vi "Dresden R2R Sputter 03.02.2018 IY24.vi"() -> ()   [LabVIEW 2009] (continued)
        n1597 = In Range and Coerce(upper limit=1002, x=w2926, lower limit=965) -> (In Range?=w3115:bool)  [unwired: 1 out]
        n1598 = In Range and Coerce(upper limit=679, x=w2926, lower limit=640) -> (In Range?=w3110:bool)  [unwired: 1 out]
        n1599 = In Range and Coerce(upper limit=475, x=w2926, lower limit=441) -> (In Range?=w3081:bool)  [unwired: 1 out]
        n1600 = In Range and Coerce(upper limit=115, x=w2925, lower limit=31) -> (In Range?=w3449:bool)  [unwired: 1 out]
        n1601 = In Range and Coerce(upper limit=537, x=w2926, lower limit=455) -> (In Range?=w3428:bool)  [unwired: 1 out]
        n1602 = In Range and Coerce(upper limit=1158, x=w2926, lower limit=1122) -> (In Range?=w3325:bool)  [unwired: 1 out]
        n1603 = In Range and Coerce(upper limit=450, x=w2925, lower limit=401) -> (In Range?=w3310:bool)  [unwired: 1 out]
        n1604 = In Range and Coerce(upper limit=440, x=w2926, lower limit=409) -> (In Range?=w3292:bool)  [unwired: 1 out]
        n1605 = In Range and Coerce(upper limit=456, x=w2925, lower limit=392) -> (In Range?=w3259:bool)  [unwired: 1 out]
        n1606 = In Range and Coerce(upper limit=537, x=w2926, lower limit=445) -> (In Range?=w3277:bool)  [unwired: 1 out]
        n1607 = In Range and Coerce(upper limit=296, x=w2925, lower limit=263) -> (In Range?=w3229:bool)  [unwired: 1 out]
        n1608 = In Range and Coerce(upper limit=492, x=w2925, lower limit=468) -> (In Range?=w3175:bool)  [unwired: 1 out]
        n1609 = In Range and Coerce(upper limit=485, x=w2925, lower limit=464) -> (In Range?=w3126:bool)  [unwired: 1 out]
        n1610 = In Range and Coerce(upper limit=1188, x=w2926, lower limit=1106) -> (In Range?=w3450:bool)  [unwired: 1 out]
        n1611 = In Range and Coerce(upper limit=1088, x=w2926, lower limit=1060) -> (In Range?=w3311:bool)  [unwired: 1 out]
        n1612 = In Range and Coerce(upper limit=1188, x=w2926, lower limit=1105) -> (In Range?=w3258:bool)  [unwired: 1 out]
        n1613 = In Range and Coerce(upper limit=296, x=w2925, lower limit=263) -> (In Range?=w3246:bool)  [unwired: 1 out]
        n1614 = In Range and Coerce(upper limit=979, x=w2926, lower limit=961) -> (In Range?=w3228:bool)  [unwired: 1 out]
        n1615 = In Range and Coerce(upper limit=296, x=w2925, lower limit=263) -> (In Range?=w3213:bool)  [unwired: 1 out]
        n1616 = In Range and Coerce(upper limit=492, x=w2925, lower limit=468) -> (In Range?=w3158:bool)  [unwired: 1 out]
        n1617 = In Range and Coerce(upper limit=433, x=w2926, lower limit=385) -> (In Range?=w3176:bool)  [unwired: 1 out]
        n1618 = In Range and Coerce(upper limit=492, x=w2925, lower limit=468) -> (In Range?=w3187:bool)  [unwired: 1 out]
        n1619 = In Range and Coerce(upper limit=485, x=w2925, lower limit=464) -> (In Range?=w3143:bool)  [unwired: 1 out]
        n1620 = In Range and Coerce(upper limit=552, x=w2926, lower limit=456) -> (In Range?=w3125:bool)  [unwired: 1 out]
        n1621 = In Range and Coerce(upper limit=685, x=w2925, lower limit=536) -> (In Range?=w3114:bool)  [unwired: 1 out]
        n1622 = In Range and Coerce(upper limit=751, x=w2925, lower limit=717) -> (In Range?=w3077:bool)  [unwired: 1 out]
        n1623 = In Range and Coerce(upper limit=328, x=w2926, lower limit=307) -> (In Range?=w3247:bool)  [unwired: 1 out]
        n1624 = In Range and Coerce(upper limit=682, x=w2926, lower limit=661) -> (In Range?=w3214:bool)  [unwired: 1 out]
        n1625 = In Range and Coerce(upper limit=1085, x=w2926, lower limit=1049) -> (In Range?=w3157:bool)  [unwired: 1 out]
        n1626 = In Range and Coerce(upper limit=597, x=w2926, lower limit=557) -> (In Range?=w3186:bool)  [unwired: 1 out]
        n1627 = In Range and Coerce(upper limit=1201, x=w2926, lower limit=1111) -> (In Range?=w3144:bool)  [unwired: 1 out]
        n1628 = In Range and Coerce(upper limit=798, x=w2926, lower limit=767) -> (In Range?=w3076:bool)  [unwired: 1 out]
        n1629 = And(x=w3410, y=w3411) -> (x .and. y?=w3389:bool)
        n1630 = And(x=w3401, y=w3400) -> (x .and. y?=w3391:bool)
        n1631 = And(x=w2958, y=w2957) -> (x .and. y?=w2776:bool)
        n1632 = And(x=w3415, y=w3414) -> (x .and. y?=w3390:bool)
        n1633 = And(x=w3371, y=w3370) -> (x .and. y?=w3357:bool)
        n1634 = And(x=w2995, y=w2996) -> (x .and. y?=w2977:bool)
        n1635 = And(x=w2943, y=w2944) -> (x .and. y?=w2923:bool)
        n1636 = And(x=w3396, y=w3397) -> (x .and. y?=w3392:bool)
        n1637 = And(x=w3380, y=w3381) -> (x .and. y?=w3359:bool)
        n1638 = And(x=w3014, y=w3013) -> (x .and. y?=w3005:bool)
        n1639 = And(x=w2955, y=w2956) -> (x .and. y?=w2775:bool)
        n1640 = And(x=w3339, y=w3340) -> (x .and. y?=w3318:bool)
        n1641 = And(x=w2998, y=w2997) -> (x .and. y?=w2978:bool)
        n1642 = And(x=w2946, y=w2945) -> (x .and. y?=w2924:bool)
        n1643 = And(x=w3433, y=w3432) -> (x .and. y?=w3422:bool)
        n1644 = And(x=w3366, y=w3367) -> (x .and. y?=w3358:bool)
        n1645 = And(x=w3330, y=w3329) -> (x .and. y?=w3320:bool)
        n1646 = And(x=w3297, y=w3296) -> (x .and. y?=w3283:bool)
        n1647 = And(x=w3272, y=w3273) -> (x .and. y?=w3251:bool)
        n1648 = And(x=w3101, y=w3100) -> (x .and. y?=w3093:bool)
        n1649 = And(x=w3090, y=w3091) -> (x .and. y?=w3060:bool)
        n1650 = And(x=w3052, y=w3053) -> (x .and. y?=w3034:bool)
        n1651 = And(x=w3011, y=w3012) -> (x .and. y?=w3006:bool)
        n1652 = And(x=w2967, y=w2968) -> (x .and. y?=w2777:bool)
        n1653 = And(x=w3443, y=w3444) -> (x .and. y?=w3438:bool)
        n1654 = And(x=w3385, y=w3384) -> (x .and. y?=w3360:bool)
        n1655 = And(x=w3306, y=w3307) -> (x .and. y?=w3285:bool)
        n1656 = And(x=w3263, y=w3262) -> (x .and. y?=w3253:bool)
        n1657 = And(x=w3233, y=w3232) -> (x .and. y?=w3219:bool)
        n1658 = And(x=w3171, y=w3172) -> (x .and. y?=w3150:bool)
        n1659 = And(x=w3130, y=w3129) -> (x .and. y?=w3096:bool)
        n1660 = And(x=w3069, y=w3070) -> (x .and. y?=w3063:bool)
        n1661 = And(x=w3055, y=w3054) -> (x .and. y?=w3035:bool)
        n1662 = And(x=w2986, y=w2985) -> (x .and. y?=w2976:bool)
        n1663 = And(x=w2934, y=w2933) -> (x .and. y?=w2773:bool)
        n1664 = And(x=w3344, y=w3343) -> (x .and. y?=w3319:bool)
        n1665 = And(x=w3242, y=w3243) -> (x .and. y?=w3221:bool)
        n1666 = And(x=w3209, y=w3210) -> (x .and. y?=w3203:bool)
        n1667 = And(x=w3162, y=w3161) -> (x .and. y?=w3152:bool)
        n1668 = And(x=w3191, y=w3190) -> (x .and. y?=w3148:bool)
        n1669 = And(x=w3139, y=w3140) -> (x .and. y?=w3031:bool)
        n1670 = And(x=w3110, y=w3111) -> (x .and. y?=w3094:bool)
        n1671 = And(x=w3081, y=w3080) -> (x .and. y?=w3061:bool)
        n1672 = And(x=w3043, y=w3042) -> (x .and. y?=w3033:bool)
        n1673 = And(x=w3023, y=w3024) -> (x .and. y?=w3004:bool)
        n1674 = And(x=w3428, y=w3429) -> (x .and. y?=w3423:bool)
        n1675 = And(x=w3325, y=w3326) -> (x .and. y?=w3321:bool)
        n1676 = And(x=w3292, y=w3293) -> (x .and. y?=w3284:bool)
        n1677 = And(x=w3277, y=w3276) -> (x .and. y?=w3252:bool)
        n1678 = And(x=w3450, y=w3449) -> (x .and. y?=w3446:bool)
        n1679 = And(x=w3311, y=w3310) -> (x .and. y?=w3286:bool)
        n1680 = And(x=w3258, y=w3259) -> (x .and. y?=w3254:bool)
        n1681 = And(x=w3228, y=w3229) -> (x .and. y?=w3220:bool)
        n1682 = And(x=w3176, y=w3175) -> (x .and. y?=w3151:bool)
        n1683 = And(x=w3125, y=w3126) -> (x .and. y?=w3097:bool)
        n1684 = And(x=w2970, y=w2969) -> (x .and. y?=w2778:bool)
        n1685 = And(x=w3247, y=w3246) -> (x .and. y?=w3222:bool)
        n1686 = And(x=w3214, y=w3213) -> (x .and. y?=w3204:bool)
        n1687 = And(x=w3157, y=w3158) -> (x .and. y?=w3153:bool)
        n1688 = And(x=w3186, y=w3187) -> (x .and. y?=w3149:bool)
        n1689 = And(x=w3144, y=w3143) -> (x .and. y?=w3098:bool)
        n1690 = And(x=w3115, y=w3114) -> (x .and. y?=w3095:bool)
        n1691 = And(x=w3076, y=w3077) -> (x .and. y?=w3062:bool)
        n1692 = And(x=w2983, y=w2984) -> (x .and. y?=w2975:bool)
        n1693 = And(x=w2931, y=w2932) -> (x .and. y?=w2774:bool)
        n1694 = And(x=w3026, y=w3025) -> (x .and. y?=w3003:bool)
        n1695 = And(x=w3040, y=w3041) -> (x .and. y?=w3032:bool)
        n1696 = And(x=w3064, y=w3392) -> (x .and. y?=w3398:bool)
        n1697 = And(x=w3064, y=w3391) -> (x .and. y?=w3399:bool)
        n1698 = And(x=w3064, y=w3390) -> (x .and. y?=w3413:bool)
        n1699 = And(x=w3064, y=w3389) -> (x .and. y?=w3412:bool)
        n1700 = And(x=w3064, y=w3360) -> (x .and. y?=w3383:bool)
        n1701 = And(x=w3064, y=w3359) -> (x .and. y?=w3382:bool)
        n1702 = And(x=w3064, y=w3358) -> (x .and. y?=w3368:bool)
        n1703 = And(x=w3064, y=w3357) -> (x .and. y?=w3369:bool)
        n1704 = And(x=w3064, y=w3321) -> (x .and. y?=w3327:bool)
        n1705 = And(x=w3064, y=w3320) -> (x .and. y?=w3328:bool)
        n1706 = And(x=w3064, y=w3319) -> (x .and. y?=w3342:bool)
        n1707 = And(x=w3064, y=w3318) -> (x .and. y?=w3341:bool)
        n1708 = And(x=w3064, y=w3446) -> (x .and. y?=w3448:bool)
        n1709 = And(x=w3064, y=w3438) -> (x .and. y?=w3445:bool)
        n1710 = And(x=w3064, y=w3423) -> (x .and. y?=w3430:bool)
        n1711 = And(x=w3064, y=w3422) -> (x .and. y?=w3431:bool)
        n1712 = And(x=w3064, y=w3286) -> (x .and. y?=w3309:bool)
        n1713 = And(x=w3064, y=w3285) -> (x .and. y?=w3308:bool)
        n1714 = And(x=w3064, y=w3284) -> (x .and. y?=w3294:bool)
        n1715 = And(x=w3064, y=w3283) -> (x .and. y?=w3295:bool)
        n1716 = And(x=w3064, y=w3254) -> (x .and. y?=w3260:bool)
        n1717 = And(x=w3064, y=w3253) -> (x .and. y?=w3261:bool)
        n1718 = And(x=w3064, y=w3252) -> (x .and. y?=w3275:bool)
        n1719 = And(x=w3064, y=w3251) -> (x .and. y?=w3274:bool)
        n1720 = And(x=w3064, y=w3093) -> (x .and. y?=w3099:bool)
        n1721 = And(x=w3064, y=w3060) -> (x .and. y?=w3092:bool)
        n1722 = And(x=w3064, y=w3222) -> (x .and. y?=w3245:bool)
        n1723 = And(x=w3064, y=w3221) -> (x .and. y?=w3244:bool)
        n1724 = And(x=w3064, y=w3220) -> (x .and. y?=w3230:bool)
        n1725 = And(x=w3064, y=w3219) -> (x .and. y?=w3231:bool)
        n1726 = And(x=w3064, y=w3153) -> (x .and. y?=w3159:bool)
        n1727 = And(x=w3064, y=w3152) -> (x .and. y?=w3160:bool)
        n1728 = And(x=w3064, y=w3151) -> (x .and. y?=w3174:bool)
        n1729 = And(x=w3064, y=w3150) -> (x .and. y?=w3173:bool)
        n1730 = And(x=w3064, y=w3098) -> (x .and. y?=w3142:bool)
        n1731 = And(x=w3064, y=w3031) -> (x .and. y?=w3141:bool)
        n1732 = And(x=w3064, y=w3097) -> (x .and. y?=w3127:bool)
        n1733 = And(x=w3064, y=w3096) -> (x .and. y?=w3128:bool)
        n1734 = And(x=w3064, y=w3063) -> (x .and. y?=w3071:bool)
        n1735 = And(x=w3064, y=w3204) -> (x .and. y?=w3212:bool)
        n1736 = And(x=w3064, y=w3203) -> (x .and. y?=w3211:bool)
        n1737 = And(x=w3064, y=w3149) -> (x .and. y?=w3188:bool)
        n1738 = And(x=w3064, y=w3148) -> (x .and. y?=w3189:bool)
        n1739 = And(x=w3064, y=w3095) -> (x .and. y?=w3113:bool)
        n1740 = And(x=w3064, y=w3094) -> (x .and. y?=w3112:bool)
        n1741 = And(x=w3064, y=w3062) -> (x .and. y?=w3078:bool)
        n1742 = And(x=w3064, y=w3061) -> (x .and. y?=w3079:bool)
        n1743 = case shown="True" w3413 {
          frame #0 {
          }
          frame #1 {
            "Ch3_Pl_vbv_timer" <- TRUE ("Mp3_timer")
          }
        }
        n1744 = case shown="True" w3412 {
          frame #0 {
          }
          frame #1 {
            "Ch4_Pl_vbv_timer" <- TRUE ("Mp4_timer")
          }
        }
        n1745 = case shown="True" w3398 {
          frame #0 {
          }
          frame #1 {
            "Ch1_Pl_vbv_timer" <- TRUE ("Mp1_timer")
          }
        }
        n1746 = case shown="True" w3399 {
          frame #0 {
          }
          frame #1 {
            "Ch2_Pl_vbv_timer" <- TRUE ("Mp2_timer")
          }
        }
        n1747 = case shown="True" w3368 {
          frame #0 {
          }
          frame #1 {
            "Ch3_Bg_bv_timer" <- TRUE ("Mp3_timer")
          }
        }
        n1748 = case shown="True" w3369 {
          frame #0 {
          }
          frame #1 {
            "Ch4_Bg_bv_timer" <- TRUE ("Mp4_timer")
          }
        }
        n1749 = case shown="True" w3342 {
          frame #0 {
          }
          frame #1 {
            "Ch3_Tp_bv_timer" <- TRUE ("Mp3_timer")
          }
        }
        n1750 = case shown="True" w3430 {
          frame #0 {
          }
          frame #1 {
            "Ch3_Mp_timer" <- TRUE ("Mp3_timer")
          }
        }
        n1751 = case shown="True" w3383 {
          frame #0 {
          }
          frame #1 {
            "Ch1_Bg_bv_timer" <- TRUE ("Mp1_timer")
          }
        }
        n1752 = case shown="True" w3382 {
          frame #0 {
          }
          frame #1 {
            "Ch2_Bg_bv_timer" <- TRUE ("Mp2_timer")
          }
        }
        n1753 = case shown="True" w3294 {
          frame #0 {
          }
          frame #1 {
            "Ch3_Ch_vbv_timer" <- TRUE ("Mp3_timer")
          }
        }
        n1754 = case shown="True" w3275 {
          frame #0 {
          }
          frame #1 {
            "Ch3_Tp_timer" <- TRUE ("Mp3_timer")
          }
        }
        n1755 = case shown="True" w3341 {
          frame #0 {
          }
          frame #1 {
            "Ch4_Tp_bv_timer" <- TRUE ("Mp4_timer")
          }
        }
        n1756 = case shown="True" w3230 {
          frame #0 {
          }
          frame #1 {
            "Bp_bv_timer_ch3_R" <- TRUE ("Mp3_timer")
          }
        }
        n1757 = case shown="True" w3174 {
          frame #0 {
          }
          frame #1 {
            "Ch3_Trns_gv_bp2" <- TRUE ("Mp3_timer")
          }
        }
        n1758 = case shown="True" w3127 {
          frame #0 {
          }
          frame #1 {
            "Ch3_Pc_bv_timer" <- TRUE ("Mp3_timer")
          }
        }
        n1759 = case shown="True" w3431 {
          frame #0 {
          }
          frame #1 {
            "Ch4_Mp_timer" <- TRUE ("Mp4_timer")
          }
        }
        n1760 = case shown="True" w3327 {
          frame #0 {
          }
          frame #1 {
            "Ch1_Tp_bv_timer" <- TRUE ("Mp1_timer")
          }
        }
        n1761 = case shown="True" w3328 {
          frame #0 {
          }
          frame #1 {
            "Ch2_Tp_bv_timer" <- TRUE ("Mp2_timer")
          }
        }
        n1762 = case shown="True" w3295 {
          frame #0 {
          }
          frame #1 {
            "Ch4_Ch_vbv_timer" <- TRUE ("Mp4_timer")
          }
        }
        n1763 = case shown="True" w3274 {
          frame #0 {
          }
          frame #1 {
            "Ch4_Tp_timer" <- TRUE ("Mp4_timer")
          }
        }
        n1764 = case shown="True" w3212 {
          frame #0 {
          }
          frame #1 {
            "Bp_bv_timer_ch3_L" <- TRUE ("Mp3_timer")
          }
        }
        n1765 = case shown="True" w3188 {
          frame #0 {
          }
          frame #1 {
            "Ch3_Trns_gv_bp" <- TRUE ("Mp3_timer")
          }
        }
        n1766 = case shown="True" w3113 {
          frame #0 {
          }
          frame #1 {
            "Gv_timer_ch1_2" <- TRUE ("Mp3_timer")
          }
        }
        n1767 = case shown="True" w3099 {
          frame #0 {
          }
          frame #1 {
            "Gv_timer_ch3_4" <- TRUE ("Mp4_timer")
          }
        }
        n1768 = case shown="True" w3078 {
          frame #0 {
          }
          frame #1 {
            "Ch2_Cc_timer" <- TRUE ("Mp3_timer")
          }
        }
        n1769 = case shown="True" w3092 {
          frame #0 {
          }
          frame #1 {
            "Ch4_Cc_timer" <- TRUE ("Mp4_timer")
          }
        }
        n1770 = case shown="True" w3448 {
          frame #0 {
          }
          frame #1 {
            "Ch1_Mp_timer" <- TRUE ("Mp1_timer")
          }
        }
        n1771 = case shown="True" w3445 {
          frame #0 {
          }
          frame #1 {
            "Ch2_Mp_timer" <- TRUE ("Mp2_timer")
          }
        }
        n1772 = case shown="True" w3309 {
          frame #0 {
          }
          frame #1 {
            "Ch1_Ch_vbv_timer" <- TRUE ("Mp1_timer")
          }
        }
        n1773 = case shown="True" w3308 {
          frame #0 {
          }
          frame #1 {
            "Ch2_Ch_vbv_timer" <- TRUE ("Mp2_timer")
          }
        }
        n1774 = case shown="True" w3260 {
          frame #0 {
          }
          frame #1 {
            "Ch1_Tp_timer" <- TRUE ("Mp1_timer")
          }
        }
        n1775 = case shown="True" w3261 {
          frame #0 {
          }
          frame #1 {
            "Ch2_Tp_timer" <- TRUE ("Mp2_timer")
          }
        }
        n1776 = case shown="True" w3231 {
          frame #0 {
          }
          frame #1 {
            "Bp_bv_timer_ch2_L" <- TRUE ("Mp4_timer")
          }
        }
        n1777 = case shown="True" w3173 {
          frame #0 {
          }
          frame #1 {
            "Ch2_Trns_gv_bp" <- TRUE ("Mp4_timer")
          }
        }
        n1778 = case shown="True" w3128 {
          frame #0 {
          }
          frame #1 {
            "Ch4_Pc_bv_timer" <- TRUE ("Mp4_timer")
          }
        }
        n1779 = case shown="True" w3071 {
          frame #0 {
          }
          frame #1 {
            "Ch1_Cc_timer" <- TRUE ("Mp4_timer")
          }
        }
        n1780 = case shown="True" w3245 {
          frame #0 {
          }
          frame #1 {
            "Bp_bv_timer_ch1_R" <- TRUE ("Mp1_timer")
          }
        }
        n1781 = case shown="True" w3244 {
          frame #0 {
          }
          frame #1 {
            "Bp_bv_timer_ch2_R" <- TRUE ("Mp2_timer")
          }
        }
        n1782 = case shown="True" w3211 {
          frame #0 {
          }
          frame #1 {
            "Bp_bv_timer_ch4_L" <- TRUE ("Mp4_timer")
          }
        }
        n1783 = case shown="True" w3159 {
          frame #0 {
          }
          frame #1 {
            "Ch1_Trns_gv_bp2" <- TRUE ("Mp1_timer")
          }
        }
        n1784 = case shown="True" w3160 {
          frame #0 {
          }
          frame #1 {
            "Ch2_Trns_gv_bp2" <- TRUE ("Mp2_timer")
          }
        }
        n1785 = case shown="True" w3189 {
          frame #0 {
          }
          frame #1 {
            "Ch4_Trns_gv_bp" <- TRUE ("Mp4_timer")
          }
        }
        n1786 = case shown="True" w3142 {
          frame #0 {
          }
          frame #1 {
            "Ch1_Pc_bv_timer" <- TRUE ("Mp1_timer")
          }
        }
        n1787 = case shown="True" w3141 {
          frame #0 {
          }
          frame #1 {
            "Ch2_Pc_bv_timer" <- TRUE ("Mp2_timer")
          }
        }
        n1788 = case shown="True" w3112 {
          frame #0 {
          }
          frame #1 {
            "Gv_timer_ch2_3" <- TRUE ("Mp4_timer")
          }
        }
        n1789 = case shown="True" w3079 {
          frame #0 {
          }
          frame #1 {
            "Ch3_Cc_timer" <- TRUE ("Mp4_timer")
          }
        }
        n1790 = Build Array(FALSE, w3446, w3438, w3423, w3422, w3392, w3391, w3390, w3389, w3360, w3359, w3358, w3357, w3321, w3320, w3319, w3318, w3286, w3285, w3284, w3283, w3254, w3253, w3252, w3251, w3222, w3221, w3220, w3219, w3204, w3203) -> (w3421:bool[])
        n1791 = Build Array(FALSE, w3153, w3152, w3151, w3150, w3149, w3148, w3098, w3031, w3097, w3096, w3095, w3094, w3093, w3063, w3062, w3061, w3060, w3035, w3034, w3033, w3032, w3006, w3005, w3004, w3003, w2978, w2977, w2976, w2975, w2924, w2923) -> (w3200:bool[])
        n1792 = Build Array(FALSE, w2773, w2774, w2775, w2776, w2777, w2778) -> (w2772:bool[])
        n1793 = Boolean Array To Number(Boolean array=w3421) -> (number=w3420:u32)
        n1794 = Boolean Array To Number(Boolean array=w3200) -> (number=w3201:u32)
        n1795 = Mantissa & Exponent(0:w3420) -> (2:w3198:dbl)  [unwired: 1 out]
        n1796 = Boolean Array To Number(Boolean array=w2772) -> (number=w2781:u32)
        n1797 = Mantissa & Exponent(0:w3201) -> (2:w3199:dbl)  [unwired: 1 out]
        n1798 = stacked-sequence {
          frame #0 {
            # "gui tab"
          }
        }
        n1799 = Mantissa & Exponent(0:w2781) -> (2:w2780:dbl)  [unwired: 1 out]
        n1800 = case shown="6" w2780 {
          tunnel: [0.0 ("y") 62.0 ("y") 63.0 ("y") 64.0 ("y") 65.0 ("y") 66.0 ("y") 67.0 ("y")] -> w2769
          frame #0 {
          }
          frame #1 {
          }
          frame #2 {
          }
          frame #3 {
          }
          frame #4 {
          }
          frame #5 {
          }
          frame #6 {
          }
        }
        n1801 = case shown="0, Default" w3199 {
          tunnel: [0 31 32 33 34 35 36 37 38 39 40 41 42 43 44 45 46 47 48 49 50 51 52 53 54 55 56 57 58 59 60 61 62 63 64 65 66 67] -> w3197
          frame #0 {
          }
          frame #1 {
          }
          frame #2 {
          }
          frame #3 {
          }
          frame #4 {
          }
          frame #5 {
          }
          frame #6 {
          }
          frame #7 {
          }
          frame #8 {
          }
          frame #9 {
          }
          frame #10 {
          }
          frame #11 {
          }
          frame #12 {
          }
          frame #13 {
          }
          frame #14 {
          }
          frame #15 {
          }
          frame #16 {
          }
          frame #17 {
          }
          frame #18 {
          }
          frame #19 {
          }
          frame #20 {
          }
          frame #21 {
          }
          frame #22 {
          }
          frame #23 {
          }
          frame #24 {
          }
          frame #25 {
          }
          frame #26 {
          }
          frame #27 {
          }
          frame #28 {
          }
          frame #29 {
          }
          frame #30 {
          }
          frame #31 {
          }
          frame #32 {
          }
          frame #33 {
          }
          frame #34 {
          }
          frame #35 {
          }
          frame #36 {
          }
          frame #37 {
          }
        }
        n1802 = local read "Ch1_Pl_vbv_timer"() -> (w2912:bool)
        n1803 = local read "Ch3_Pl_vbv_timer"() -> (w2910:bool)
        n1804 = local read "Ch4_Pl_vbv_timer"() -> (w2909:bool)
        n1805 = local read "Ch3_Mp_timer"() -> (w2914:bool)
        n1806 = local read "Ch2_Pl_vbv_timer"() -> (w2911:bool)
        n1807 = local read "Ch2_Mp_timer"() -> (w2919:bool)
        n1808 = local read "Ch1_Bg_bv_timer"() -> (w2896:bool)
        n1809 = local read "Ch1_Mp_timer"() -> (w2920:bool)
        n1810 = local read "Ch4_Mp_timer"() -> (w2913:bool)
        n1811 = local read "Ch2_Bg_bv_timer"() -> (w2895:bool)
        n1812 = local read "Ch1_Tp_bv_timer"() -> (w2884:bool)
        n1813 = local read "Ch3_Bg_bv_timer"() -> (w2890:bool)
        n1814 = local read "Ch4_Bg_bv_timer"() -> (w2889:bool)
        n1815 = local read "Ch2_Tp_bv_timer"() -> (w2883:bool)
        n1816 = local read "Ch3_Tp_bv_timer"() -> (w2878:bool)
        n1817 = local read "Ch1_Ch_vbv_timer"() -> (w2872:bool)
        n1818 = local read "Ch4_Tp_bv_timer"() -> (w2877:bool)
        n1819 = local read "Ch2_Pc_bv_timer"() -> (w2847:bool)
        n1820 = local read "Ch2_Ch_vbv_timer"() -> (w2871:bool)
        n1821 = local read "Ch4_Ch_vbv_timer"() -> (w2865:bool)
        n1822 = local read "Ch3_Pc_bv_timer"() -> (w2842:bool)
        n1823 = local read "Ch3_Ch_vbv_timer"() -> (w2866:bool)
        n1824 = local read "Ch1_Pc_bv_timer"() -> (w2848:bool)
        n1825 = local read "Ch4_Pc_bv_timer"() -> (w2841:bool)
        n1826 = local read "Ch2_Trns_gv_bp2"() -> (w2794:bool)
        n1827 = local read "Gv_timer_ch1_2"() -> (w2836:bool)
        n1828 = local read "Ch4_Tp_timer"() -> (w2853:bool)
        n1829 = local read "Gv_timer_ch2_3"() -> (w2835:bool)
        n1830 = local read "Ch3_Tp_timer"() -> (w2854:bool)
        n1831 = local read "Gv_timer_ch3_4"() -> (w2830:bool)
        n1832 = local read "Ch1_Tp_timer"() -> (w2860:bool)
        n1833 = local read "Ch2_Tp_timer"() -> (w2859:bool)
        n1834 = local read "Bp_bv_timer_ch1_R"() -> (w2817:bool)
        n1835 = local read "Ch1_Cc_timer"() -> (w2829:bool)
        n1836 = local read "Bp_bv_timer_ch3_R"() -> (w2811:bool)
        n1837 = local read "Bp_bv_timer_ch3_L"() -> (w2805:bool)
        n1838 = local read "Bp_bv_timer_ch4_L"() -> (w2800:bool)
        n1839 = local read "Ch3_Trns_gv_bp2"() -> (w2793:bool)
        n1840 = local read "Bp_bv_timer_ch2_R"() -> (w2812:bool)
        n1841 = local read "Bp_bv_timer_ch2_L"() -> (w2806:bool)
        n1842 = local read "Ch1_Trns_gv_bp2"() -> (w2799:bool)
        n1843 = local read "Ch3_Cc_timer"() -> (w2823:bool)
        n1844 = local read "Ch2_Trns_gv_bp"() -> (w2788:bool)
        n1845 = Add(x=w3198, y=w3197) -> (x+y=w2768:dbl)
        n1846 = local read "Ch2_Cc_timer"() -> (w2824:bool)
        n1847 = local read "Ch3_Trns_gv_bp"() -> (w2787:bool)
        n1848 = feedback #7() -> (w2916:bool)  [unwired: 1 in]
        n1849 = feedback #8() -> (w2917:bool)  [unwired: 1 in]
        n1850 = local read "Ch4_Cc_timer"() -> (w2818:bool)
        n1851 = local read "Ch4_Trns_gv_bp"() -> (w2782:bool)
        n1852 = feedback #9() -> (w2922:bool)  [unwired: 1 in]
        n1853 = feedback #10() -> (w2907:bool)  [unwired: 1 in]
        n1854 = feedback #11() -> (w2905:bool)  [unwired: 1 in]
        n1855 = feedback #12() -> (w2901:bool)  [unwired: 1 in]
        n1856 = feedback #13() -> (w2899:bool)  [unwired: 1 in]
        n1857 = feedback #14() -> (w2903:bool)  [unwired: 1 in]
        n1858 = feedback #15() -> (w2898:bool)  [unwired: 1 in]
        n1859 = feedback #16() -> (w2893:bool)  [unwired: 1 in]
        n1860 = feedback #17() -> (w2886:bool)  [unwired: 1 in]
        n1861 = feedback #18() -> (w2892:bool)  [unwired: 1 in]
        n1862 = feedback #19() -> (w2887:bool)  [unwired: 1 in]
        n1863 = feedback #20() -> (w2881:bool)  [unwired: 1 in]
        n1864 = feedback #21() -> (w2880:bool)  [unwired: 1 in]
        n1865 = feedback #22() -> (w2875:bool)  [unwired: 1 in]
        n1866 = feedback #23() -> (w2845:bool)  [unwired: 1 in]
        n1867 = feedback #24() -> (w2844:bool)  [unwired: 1 in]
        n1868 = feedback #25() -> (w2874:bool)  [unwired: 1 in]
        n1869 = feedback #26() -> (w2850:bool)  [unwired: 1 in]
        n1870 = feedback #27() -> (w2839:bool)  [unwired: 1 in]
        n1871 = feedback #28() -> (w2851:bool)  [unwired: 1 in]
        n1872 = feedback #29() -> (w2869:bool)  [unwired: 1 in]
        n1873 = feedback #30() -> (w2863:bool)  [unwired: 1 in]
        n1874 = feedback #31() -> (w2856:bool)  [unwired: 1 in]
        n1875 = feedback #32() -> (w2868:bool)  [unwired: 1 in]
        n1876 = feedback #33() -> (w2862:bool)  [unwired: 1 in]
        n1877 = feedback #34() -> (w2838:bool)  [unwired: 1 in]
        n1878 = feedback #35() -> (w2857:bool)  [unwired: 1 in]
        n1879 = feedback #36() -> (w2833:bool)  [unwired: 1 in]
        n1880 = feedback #37() -> (w2827:bool)  [unwired: 1 in]
        n1881 = feedback #38() -> (w2832:bool)  [unwired: 1 in]
        n1882 = feedback #39() -> (w2821:bool)  [unwired: 1 in]
        n1883 = feedback #40() -> (w2826:bool)  [unwired: 1 in]
        n1884 = feedback #41() -> (w2820:bool)  [unwired: 1 in]
        n1885 = feedback #42() -> (w2791:bool)  [unwired: 1 in]
        n1886 = feedback #43() -> (w2796:bool)  [unwired: 1 in]
        n1887 = feedback #44() -> (w2790:bool)  [unwired: 1 in]
        n1888 = feedback #45() -> (w2815:bool)  [unwired: 1 in]
        n1889 = feedback #46() -> (w2785:bool)  [unwired: 1 in]
        n1890 = feedback #47() -> (w2809:bool)  [unwired: 1 in]
        n1891 = feedback #48() -> (w2803:bool)  [unwired: 1 in]
        n1892 = feedback #49() -> (w2797:bool)  [unwired: 1 in]
        n1893 = feedback #50() -> (w2802:bool)  [unwired: 1 in]
        n1894 = feedback #51() -> (w2784:bool)  [unwired: 1 in]
        n1895 = feedback #52() -> (w2814:bool)  [unwired: 1 in]
        n1896 = feedback #53() -> (w2808:bool)  [unwired: 1 in]
        n1897 = case shown="True" w2914 {
          tunnel: w2916 -> [_ w3916]
          tunnel: [TRUE FALSE] -> w2915
          frame #0 {
          }
          frame #1 {
            n1898 = call "Elapsed Time3"("Reset"=w3916) -> ("Elapsed Time (s)"=w3915:dbl)  [unwired: 11 in, 7 out]
            n1899 = Greater?(x=w3915, y=3.0) -> (0:w3922:bool)
            n1900 = Not(x=w3922) -> (.not. x?=w3918:bool)
            n1901 = In Range and Coerce(upper limit=3.0, x=w3915, lower limit=0.0) -> (In Range?=w3914:bool)  [unwired: 1 out]
            n1902 = local write "Ch3_Mp_timer"(w3918) -> ()
            n1903 = property on="Mp_ch3_tab_gui" class="TabCtl (strict)"("Visible"=w3914) -> ()  [unwired: 2 in, 2 out]
          }
        }
        n1904 = case shown="True" w2919 {
          tunnel: w2917 -> [_ w3926]
          tunnel: [TRUE FALSE] -> w2918
          frame #0 {
          }
          frame #1 {
            n1905 = call "Elapsed Time2"("Reset"=w3926) -> ("Elapsed Time (s)"=w3925:dbl)  [unwired: 11 in, 7 out]
            n1906 = Greater?(x=w3925, y=3.0) -> (0:w3932:bool)
            n1907 = Not(x=w3932) -> (.not. x?=w3928:bool)
            n1908 = In Range and Coerce(upper limit=3.0, x=w3925, lower limit=0.0) -> (In Range?=w3924:bool)  [unwired: 1 out]
            n1909 = local write "Ch2_Mp_timer"(w3928) -> ()
            n1910 = property on="Mp_ch2_tab_gui" class="TabCtl (strict)"("Visible"=w3924) -> ()  [unwired: 2 in, 2 out]
          }
        }
        n1911 = Not Equal To 0?(x=w2768) -> (x != 0?=w3196:bool)
        n1912 = case shown="True" w2920 {
          tunnel: w2922 -> [_ w3935]
          tunnel: [TRUE FALSE] -> w2921
          frame #0 {
          }
          frame #1 {
            n1913 = call "Elapsed Time"("Reset"=w3935) -> ("Elapsed Time (s)"=w3934:dbl)  [unwired: 11 in, 7 out]
            n1914 = Greater?(x=w3934, y=3.0) -> (0:w3942:bool)
            n1915 = Not(x=w3942) -> (.not. x?=w3937:bool)
            n1916 = In Range and Coerce(upper limit=3.0, x=w3934, lower limit=0.0) -> (In Range?=w3938:bool)  [unwired: 1 out]
            n1917 = local write "Ch1_Mp_timer"(w3937) -> ()
            n1918 = property on="Mp_ch1tab_gui" class="TabCtl (strict)"("Visible"=w3938) -> ()  [unwired: 2 in, 2 out]
          }
        }
        n1919 = case shown="True" w2913 {
          tunnel: w2907 -> [_ w3906]
          tunnel: [TRUE FALSE] -> w2908
          frame #0 {
          }
          frame #1 {
            n1920 = call "Elapsed Time4"("Reset"=w3906) -> ("Elapsed Time (s)"=w3905:dbl)  [unwired: 11 in, 7 out]
            n1921 = Greater?(x=w3905, y=3.0) -> (0:w3912:bool)
            n1922 = Not(x=w3912) -> (.not. x?=w3908:bool)
            n1923 = In Range and Coerce(upper limit=3.0, x=w3905, lower limit=0.0) -> (In Range?=w3904:bool)  [unwired: 1 out]
            n1924 = local write "Ch4_Mp_timer"(w3908) -> ()
            n1925 = property on="Mp_ch4_tab_gui" class="TabCtl (strict)"("Visible"=w3904) -> ()  [unwired: 2 in, 2 out]
          }
        }
        n1926 = case shown="True" w2912 {
          tunnel: w2905 -> [_ w3896]
          tunnel: [TRUE FALSE] -> w2906
          frame #0 {
          }
          frame #1 {
            n1927 = call "Elapsed Time5"("Reset"=w3896) -> ("Elapsed Time (s)"=w3895:dbl)  [unwired: 11 in, 7 out]
            n1928 = Greater?(x=w3895, y=3.0) -> (0:w3902:bool)
            n1929 = Not(x=w3902) -> (.not. x?=w3898:bool)
            n1930 = In Range and Coerce(upper limit=3.0, x=w3895, lower limit=0.0) -> (In Range?=w3894:bool)  [unwired: 1 out]
            n1931 = local write "Ch1_Pl_vbv_timer"(w3898) -> ()
            n1932 = property on="Pl_vbv_tab_ch1_gui" class="TabCtl (strict)"("Visible"=w3894) -> ()  [unwired: 2 in, 2 out]
          }
        }
        n1933 = case shown="True" w2910 {
          tunnel: w2901 -> [_ w3876]
          tunnel: [TRUE FALSE] -> w2902
          frame #0 {
          }
          frame #1 {
            n1934 = call "Elapsed Time7"("Reset"=w3876) -> ("Elapsed Time (s)"=w3875:dbl)  [unwired: 11 in, 7 out]
            n1935 = Greater?(x=w3875, y=3.0) -> (0:w3882:bool)
            n1936 = Not(x=w3882) -> (.not. x?=w3878:bool)
            n1937 = In Range and Coerce(upper limit=3.0, x=w3875, lower limit=0.0) -> (In Range?=w3874:bool)  [unwired: 1 out]
            n1938 = local write "Ch3_Pl_vbv_timer"(w3878) -> ()
            n1939 = property on="Pl_vbv_ch3_tab_gui" class="TabCtl (strict)"("Visible"=w3874) -> ()  [unwired: 2 in, 2 out]
          }
        }
        n1940 = case shown="True" w2909 {
          tunnel: w2899 -> [_ w3866]
          tunnel: [TRUE FALSE] -> w2900
          frame #0 {
          }
          frame #1 {
            n1941 = call "Elapsed Time8"("Reset"=w3866) -> ("Elapsed Time (s)"=w3865:dbl)  [unwired: 11 in, 7 out]
            n1942 = Greater?(x=w3865, y=3.0) -> (0:w3872:bool)
            n1943 = Not(x=w3872) -> (.not. x?=w3868:bool)
            n1944 = In Range and Coerce(upper limit=3.0, x=w3865, lower limit=0.0) -> (In Range?=w3864:bool)  [unwired: 1 out]
            n1945 = local write "Ch4_Pl_vbv_timer"(w3868) -> ()
            n1946 = property on="Pl_vbv_ch4_tab_gui" class="TabCtl (strict)"("Visible"=w3864) -> ()  [unwired: 2 in, 2 out]
          }
        }
        n1947 = case shown="True" w2911 {
          tunnel: w2903 -> [_ w3886]
          tunnel: [TRUE FALSE] -> w2904
          frame #0 {
          }
          frame #1 {
            n1948 = call "Elapsed Time6"("Reset"=w3886) -> ("Elapsed Time (s)"=w3885:dbl)  [unwired: 11 in, 7 out]
            n1949 = Greater?(x=w3885, y=3.0) -> (0:w3892:bool)
            n1950 = Not(x=w3892) -> (.not. x?=w3888:bool)
            n1951 = In Range and Coerce(upper limit=3.0, x=w3885, lower limit=0.0) -> (In Range?=w3884:bool)  [unwired: 1 out]
            n1952 = local write "Ch2_Pl_vbv_timer"(w3888) -> ()
            n1953 = property on="Pl_vbv_ch2_tab_gui" class="TabCtl (strict)"("Visible"=w3884) -> ()  [unwired: 2 in, 2 out]
          }
        }
        n1954 = case shown="True" w2896 {
          tunnel: w2898 -> [_ w3856]
          tunnel: [TRUE FALSE] -> w2897
          frame #0 {
          }
          frame #1 {
            n1955 = call "Elapsed Time9"("Reset"=w3856) -> ("Elapsed Time (s)"=w3855:dbl)  [unwired: 11 in, 7 out]
            n1956 = Greater?(x=w3855, y=3.0) -> (0:w3862:bool)
            n1957 = Not(x=w3862) -> (.not. x?=w3858:bool)
            n1958 = In Range and Coerce(upper limit=3.0, x=w3855, lower limit=0.0) -> (In Range?=w3854:bool)  [unwired: 1 out]
            n1959 = local write "Ch1_Bg_bv_timer"(w3858) -> ()
            n1960 = property on="Bg_bv_tab_ch1_gui" class="TabCtl (strict)"("Visible"=w3854) -> ()  [unwired: 2 in, 2 out]
          }
        }
        n1961 = case shown="True" w2895 {
          tunnel: w2893 -> [_ w3846]
          tunnel: [TRUE FALSE] -> w2894
          frame #0 {
          }
          frame #1 {
            n1962 = call "Elapsed Time10"("Reset"=w3846) -> ("Elapsed Time (s)"=w3845:dbl)  [unwired: 11 in, 7 out]
            n1963 = Greater?(x=w3845, y=3.0) -> (0:w3852:bool)
            n1964 = Not(x=w3852) -> (.not. x?=w3848:bool)
            n1965 = In Range and Coerce(upper limit=3.0, x=w3845, lower limit=0.0) -> (In Range?=w3844:bool)  [unwired: 1 out]
            n1966 = local write "Ch2_Bg_bv_timer"(w3848) -> ()
            n1967 = property on="Bg_bv_tab_ch2_gui" class="TabCtl (strict)"("Visible"=w3844) -> ()  [unwired: 2 in, 2 out]
          }
        }
        n1968 = case shown="True" w2884 {
          tunnel: w2886 -> [_ w3816]
          tunnel: [TRUE FALSE] -> w2885
          frame #0 {
          }
          frame #1 {
            n1969 = call "Elapsed Time13"("Reset"=w3816) -> ("Elapsed Time (s)"=w3815:dbl)  [unwired: 11 in, 7 out]
            n1970 = Greater?(x=w3815, y=3.0) -> (0:w3822:bool)
            n1971 = Not(x=w3822) -> (.not. x?=w3818:bool)
            n1972 = In Range and Coerce(upper limit=3.0, x=w3815, lower limit=0.0) -> (In Range?=w3814:bool)  [unwired: 1 out]
            n1973 = local write "Ch1_Tp_bv_timer"(w3818) -> ()
            n1974 = property on="Tp_bv_tab_ch1_gui" class="TabCtl (strict)"("Visible"=w3814) -> ()  [unwired: 2 in, 2 out]
          }
        }
        n1975 = case shown="True" w2890 {
          tunnel: w2892 -> [_ w3836]
          tunnel: [TRUE FALSE] -> w2891
          frame #0 {
          }
          frame #1 {
            n1976 = call "Elapsed Time11"("Reset"=w3836) -> ("Elapsed Time (s)"=w3835:dbl)  [unwired: 11 in, 7 out]
            n1977 = Greater?(x=w3835, y=3.0) -> (0:w3842:bool)
            n1978 = Not(x=w3842) -> (.not. x?=w3838:bool)
            n1979 = In Range and Coerce(upper limit=3.0, x=w3835, lower limit=0.0) -> (In Range?=w3834:bool)  [unwired: 1 out]
            n1980 = local write "Ch3_Bg_bv_timer"(w3838) -> ()
            n1981 = property on="Bg_bv_tab_ch3_gui" class="TabCtl (strict)"("Visible"=w3834) -> ()  [unwired: 2 in, 2 out]
          }
        }
        n1982 = case shown="True" w2889 {
          tunnel: w2887 -> [_ w3826]
          tunnel: [TRUE FALSE] -> w2888
          frame #0 {
          }
          frame #1 {
            n1983 = call "Elapsed Time12"("Reset"=w3826) -> ("Elapsed Time (s)"=w3825:dbl)  [unwired: 11 in, 7 out]
            n1984 = Greater?(x=w3825, y=3.0) -> (0:w3832:bool)
            n1985 = Not(x=w3832) -> (.not. x?=w3828:bool)
            n1986 = In Range and Coerce(upper limit=3.0, x=w3825, lower limit=0.0) -> (In Range?=w3824:bool)  [unwired: 1 out]
            n1987 = local write "Ch4_Bg_bv_timer"(w3828) -> ()
            n1988 = property on="Bg_bv_tab_ch1_gui 4" class="TabCtl (strict)"("Visible"=w3824) -> ()  [unwired: 2 in, 2 out]
          }
        }
        n1989 = case shown="True" w2883 {
          tunnel: w2881 -> [_ w3806]
          tunnel: [TRUE FALSE] -> w2882
          frame #0 {
          }
          frame #1 {
            n1990 = call "Elapsed Time14"("Reset"=w3806) -> ("Elapsed Time (s)"=w3805:dbl)  [unwired: 11 in, 7 out]
            n1991 = Greater?(x=w3805, y=3.0) -> (0:w3812:bool)
            n1992 = Not(x=w3812) -> (.not. x?=w3808:bool)
            n1993 = In Range and Coerce(upper limit=3.0, x=w3805, lower limit=0.0) -> (In Range?=w3804:bool)  [unwired: 1 out]
            n1994 = local write "Ch2_Tp_bv_timer"(w3808) -> ()
            n1995 = property on="Tp_bv_tab_ch2_gui" class="TabCtl (strict)"("Visible"=w3804) -> ()  [unwired: 2 in, 2 out]
          }
        }
        n1996 = case shown="True" w2878 {
          tunnel: w2880 -> [_ w3796]
          tunnel: [TRUE FALSE] -> w2879
          frame #0 {
          }
          frame #1 {
            n1997 = call "Elapsed Time15"("Reset"=w3796) -> ("Elapsed Time (s)"=w3795:dbl)  [unwired: 11 in, 7 out]
            n1998 = Greater?(x=w3795, y=3.0) -> (0:w3802:bool)
            n1999 = Not(x=w3802) -> (.not. x?=w3798:bool)
            n2000 = In Range and Coerce(upper limit=3.0, x=w3795, lower limit=0.0) -> (In Range?=w3794:bool)  [unwired: 1 out]
            n2001 = local write "Ch3_Tp_bv_timer"(w3798) -> ()
            n2002 = property on="Tp_bv_tab_ch3_gui" class="TabCtl (strict)"("Visible"=w3794) -> ()  [unwired: 2 in, 2 out]
          }
        }
        n2003 = case shown="True" w2877 {
          tunnel: w2875 -> [_ w3786]
          tunnel: [TRUE FALSE] -> w2876
          frame #0 {
          }
          frame #1 {
            n2004 = call "Elapsed Time16"("Reset"=w3786) -> ("Elapsed Time (s)"=w3785:dbl)  [unwired: 11 in, 7 out]
            n2005 = Greater?(x=w3785, y=3.0) -> (0:w3792:bool)
            n2006 = Not(x=w3792) -> (.not. x?=w3788:bool)
            n2007 = In Range and Coerce(upper limit=3.0, x=w3785, lower limit=0.0) -> (In Range?=w3784:bool)  [unwired: 1 out]
            n2008 = local write "Ch4_Tp_bv_timer"(w3788) -> ()
            n2009 = property on="Tp_bv_tab_ch4_gui" class="TabCtl (strict)"("Visible"=w3784) -> ()  [unwired: 2 in, 2 out]
          }
        }
        n2010 = case shown="True" w2847 {
          tunnel: w2845 -> [_ w3686]
          tunnel: [TRUE FALSE] -> w2846
          frame #0 {
          }
          frame #1 {
            n2011 = call "Elapsed Time26"("Reset"=w3686) -> ("Elapsed Time (s)"=w3685:dbl)  [unwired: 11 in, 7 out]
            n2012 = Greater?(x=w3685, y=3.0) -> (0:w3692:bool)
            n2013 = Not(x=w3692) -> (.not. x?=w3688:bool)
            n2014 = In Range and Coerce(upper limit=3.0, x=w3685, lower limit=0.0) -> (In Range?=w3684:bool)  [unwired: 1 out]
            n2015 = local write "Ch2_Pc_bv_timer"(w3688) -> ()
            n2016 = property on="Pc_bv_tab_ch2_gui" class="TabCtl (strict)"("Visible"=w3684) -> ()  [unwired: 2 in, 2 out]
          }
        }
        n2017 = case shown="True" w2842 {
          tunnel: w2844 -> [_ w3676]
          tunnel: [TRUE FALSE] -> w2843
          frame #0 {
          }
          frame #1 {
            n2018 = call "Elapsed Time27"("Reset"=w3676) -> ("Elapsed Time (s)"=w3675:dbl)  [unwired: 11 in, 7 out]
            n2019 = Greater?(x=w3675, y=3.0) -> (0:w3682:bool)
            n2020 = Not(x=w3682) -> (.not. x?=w3678:bool)
            n2021 = In Range and Coerce(upper limit=3.0, x=w3675, lower limit=0.0) -> (In Range?=w3674:bool)  [unwired: 1 out]
            n2022 = local write "Ch3_Pc_bv_timer"(w3678) -> ()
            n2023 = property on="Pc_bv_tab_ch3_gui" class="TabCtl (strict)"("Visible"=w3674) -> ()  [unwired: 2 in, 2 out]
          }
        }
        n2024 = case shown="True" w2872 {
          tunnel: w2874 -> [_ w3776]
          tunnel: [TRUE FALSE] -> w2873
          frame #0 {
          }
          frame #1 {
            n2025 = call "Elapsed Time17"("Reset"=w3776) -> ("Elapsed Time (s)"=w3775:dbl)  [unwired: 11 in, 7 out]
            n2026 = Greater?(x=w3775, y=3.0) -> (0:w3782:bool)
            n2027 = Not(x=w3782) -> (.not. x?=w3778:bool)
            n2028 = In Range and Coerce(upper limit=3.0, x=w3775, lower limit=0.0) -> (In Range?=w3774:bool)  [unwired: 1 out]
            n2029 = local write "Ch1_Ch_vbv_timer"(w3778) -> ()
            n2030 = property on="Ch_vbv_tab_ch1_gui" class="TabCtl (strict)"("Visible"=w3774) -> ()  [unwired: 2 in, 2 out]
          }
        }
        n2031 = case shown="True" w2848 {
          tunnel: w2850 -> [_ w3696]
          tunnel: [TRUE FALSE] -> w2849
          frame #0 {
          }
          frame #1 {
            n2032 = call "Elapsed Time25"("Reset"=w3696) -> ("Elapsed Time (s)"=w3695:dbl)  [unwired: 11 in, 7 out]
            n2033 = Greater?(x=w3695, y=3.0) -> (0:w3702:bool)
            n2034 = Not(x=w3702) -> (.not. x?=w3698:bool)
            n2035 = In Range and Coerce(upper limit=3.0, x=w3695, lower limit=0.0) -> (In Range?=w3694:bool)  [unwired: 1 out]
            n2036 = local write "Ch1_Pc_bv_timer"(w3698) -> ()
            n2037 = property on="Pc_bv_tab_ch1_gui" class="TabCtl (strict)"("Visible"=w3694) -> ()  [unwired: 2 in, 2 out]
          }
        }
        n2038 = case shown="True" w2841 {
          tunnel: w2839 -> [_ w3666]
          tunnel: [TRUE FALSE] -> w2840
          frame #0 {
          }
          frame #1 {
            n2039 = call "Elapsed Time28"("Reset"=w3666) -> ("Elapsed Time (s)"=w3665:dbl)  [unwired: 11 in, 7 out]
            n2040 = Greater?(x=w3665, y=3.0) -> (0:w3672:bool)
            n2041 = Not(x=w3672) -> (.not. x?=w3668:bool)
            n2042 = In Range and Coerce(upper limit=3.0, x=w3665, lower limit=0.0) -> (In Range?=w3664:bool)  [unwired: 1 out]
            n2043 = local write "Ch4_Pc_bv_timer"(w3668) -> ()
            n2044 = property on="Pc_bv_tab_ch4_gui" class="TabCtl (strict)"("Visible"=w3664) -> ()  [unwired: 2 in, 2 out]
          }
        }
        n2045 = case shown="True" w2853 {
          tunnel: w2851 -> [_ w3706]
          tunnel: [TRUE FALSE] -> w2852
          frame #0 {
          }
          frame #1 {
            n2046 = call "Elapsed Time24"("Reset"=w3706) -> ("Elapsed Time (s)"=w3705:dbl)  [unwired: 11 in, 7 out]
            n2047 = Greater?(x=w3705, y=3.0) -> (0:w3712:bool)
            n2048 = Not(x=w3712) -> (.not. x?=w3708:bool)
            n2049 = In Range and Coerce(upper limit=3.0, x=w3705, lower limit=0.0) -> (In Range?=w3704:bool)  [unwired: 1 out]
            n2050 = local write "Ch4_Tp_timer"(w3708) -> ()
            n2051 = property on="Tp_ch4_tab_gui" class="TabCtl (strict)"("Visible"=w3704) -> ()  [unwired: 2 in, 2 out]
          }
        }
        n2052 = case shown="True" w2871 {
          tunnel: w2869 -> [_ w3766]
          tunnel: [TRUE FALSE] -> w2870
          frame #0 {
          }
          frame #1 {
            n2053 = call "Elapsed Time18"("Reset"=w3766) -> ("Elapsed Time (s)"=w3765:dbl)  [unwired: 11 in, 7 out]